vi "neuKLEIN.vi"() -> ()   [LabVIEW 2016] (continued)
  in  "Red 88 Waveform Graph":waveform(dbl)[](graph)=[{"t0"=timestamp(0 s since 1904-01-01), "dt"=0.0001220703125, "Y"=array[4095 elements]}, {"t0"=timestamp(0 s since 1904-01-01), "dt"=0.0001220703125, "Y"=array[4095 elements]}, {"t0"=timestamp(0 s since 1904-01-01), "dt"=0.0001220703125, "Y"=array[4095 elements]}, {"t0"=timestamp(0 s since 1904-01-01), "dt"=0.0001220703125, "Y"=array[4095 elements]}]
  in  "Red MOT 88 Inputs":T21={"Active Device"="6733_Red_88", "Active Channels"=[TRUE, TRUE, TRUE, TRUE, FALSE, FALSE, FALSE, FALSE], "Waveform Parameters"=[[{"Function"=enum."Polynomial", "Initial"=-1.25, "Final"=-0.6, "Degree"=1.0, "Nickname"="Center Freq. [MHz] (0)", "Conversion"=enum."Red Boson Cntr Freq (MHz)", "Constant"=-81.284}, {"Function"=enum."Polynomial", "Initial"=-0.6, "Final"=-0.225, "Degree"=1.0, "Nickname"="(0)", "Conversion"=enum."Red Boson Cntr Freq (MHz)", "Constant"=-81.284}, {"Function"=enum."Polynomial", "Initial"=5.0, "Final"=5.0, "Degree"=1.0, "Nickname"="(0)", "Conversion"=enum."Red Boson Cntr Freq (MHz)", "Constant"=-81.284}, {"Function"=enum."Exponential", "Initial"=1.0, "Final"=0.0, "Degree"=1.0, "Nickname"="", "Conversion"=enum."B Field Grad (G/cm)", "Constant"=0.0}], [{"Function"=enum."Polynomial", "Initial"=1000.0, "Final"=550.0, "Degree"=1.0, "Nickname"="Dither Amp. [kHz] (1)", "Conversion"=enum."Red Boson Dither Amp (kHz)", "Constant"=0.0}, {"Function"=enum."Polynomial", "Initial"=550.0, "Final"=100.0, "Degree"=1.0, "Nickname"="(1)", "Conversion"=enum."Red Boson Dither Amp (kHz)", "Constant"=0.0}, {"Function"=enum."Polynomial", "Initial"=0.0, "Final"=0.0, "Degree"=1.0, "Nickname"="(1)", "Conversion"=enum."Red Boson Dither Amp (kHz)", "Constant"=0.0}, {"Function"=enum."Exponential", "Initial"=0.0, "Final"=0.0, "Degree"=1.0, "Nickname"="", "Conversion"=enum."B Field Grad (G/cm)", "Constant"=0.0}], [{"Function"=enum."Polynomial", "Initial"=10.0, "Final"=10.0, "Degree"=1.0, "Nickname"="Red Boson Power {mW} (2)", "Conversion"=enum."Red Boson Power (mW)", "Constant"=0.0}, {"Function"=enum."Polynomial", "Initial"=10.0, "Final"=5.0, "Degree"=1.0, "Nickname"="(2)", "Conversion"=enum."Red Boson Power (mW)", "Constant"=0.0}, {"Function"=enum."Exponential", "Initial"=5.0, "Final"=0.25, "Degree"=1.0, "Nickname"="(2)", "Conversion"=enum."Red Boson Power (mW)", "Constant"=0.0}, {"Function"=enum."Exponential", "Initial"=0.5, "Final"=0.5, "Degree"=1.0, "Nickname"="", "Conversion"=enum."Red Boson Power (mW)", "Constant"=0.0}], [{"Function"=enum."Polynomial", "Initial"=0.1, "Final"=1.0, "Degree"=1.0, "Nickname"="Red B-Field Grad [G/cm] (3)", "Conversion"=enum."B Field Grad (G/cm)", "Constant"=0.0}, {"Function"=enum."Polynomial", "Initial"=1.0, "Final"=2.0, "Degree"=1.0, "Nickname"="(3)", "Conversion"=enum."B Field Grad (G/cm)", "Constant"=0.0}, {"Function"=enum."Polynomial", "Initial"=2.0, "Final"=2.0, "Degree"=1.0, "Nickname"="(3)", "Conversion"=enum."B Field Grad (G/cm)", "Constant"=0.0}, {"Function"=enum."Exponential", "Initial"=0.2, "Final"=0.2, "Degree"=1.0, "Nickname"="", "Conversion"=enum."B Field Grad (G/cm)", "Constant"=0.0}], [{"Function"=enum."Constant", "Initial"=0.0, "Final"=0.0, "Degree"=1.0, "Nickname"="UNRELIABLE", "Conversion"=enum."Volts", "Constant"=0.0}, {"Function"=enum."Constant", "Initial"=0.0, "Final"=0.0, "Degree"=1.0, "Nickname"="(4)", "Conversion"=enum."Volts", "Constant"=0.0}, {"Function"=enum."Constant", "Initial"=0.0, "Final"=0.0, "Degree"=1.0, "Nickname"="(4)", "Conversion"=enum."Volts", "Constant"=0.0}, {"Function"=enum."Exponential", "Initial"=0.0, "Final"=0.0, "Degree"=1.0, "Nickname"="", "Conversion"=enum."B Field Grad (G/cm)", "Constant"=0.0}], [{"Function"=enum."Constant", "Initial"=0.0, "Final"=0.0, "Degree"=1.0, "Nickname"="Unassigned", "Conversion"=enum."Volts", "Constant"=0.0}, {"Function"=enum."Constant", "Initial"=0.0, "Final"=0.0, "Degree"=1.0, "Nickname"="(5)", "Conversion"=enum."Volts", "Constant"=0.0}, {"Function"=enum."Constant", "Initial"=0.0, "Final"=0.0, "Degree"=1.0, "Nickname"="(5)", "Conversion"=enum."Volts", "Constant"=0.0}, {"Function"=enum."Exponential", "Initial"=0.0, "Final"=0.0, "Degree"=1.0, "Nickname"="", "Conversion"=enum."B Field Grad (G/cm)", "Constant"=0.0}], [{"Function"=enum."Constant", "Initial"=0.0, "Final"=0.0, "Degree"=1.0, "Nickname"="Unassigned", "Conversion"=enum."Volts", "Constant"=0.0}, {"Function"=enum."Constant", "Initial"=0.0, "Final"=0.0, "Degree"=1.0, "Nickname"="(6)", "Conversion"=enum."Volts", "Constant"=0.0}, {"Function"=enum."Constant", "Initial"=0.0, "Final"=0.0, "Degree"=1.0, "Nickname"="(6)", "Conversion"=enum."Volts", "Constant"=0.0}, {"Function"=enum."Exponential", "Initial"=0.0, "Final"=0.0, "Degree"=1.0, "Nickname"="", "Conversion"=enum."B Field Grad (G/cm)", "Constant"=0.0}], [{"Function"=enum."Constant", "Initial"=0.0, "Final"=0.0, "Degree"=1.0, "Nickname"="Unassigned", "Conversion"=enum."Volts", "Constant"=0.0}, {"Function"=enum."Constant", "Initial"=0.0, "Final"=0.0, "Degree"=1.0, "Nickname"="(7)", "Conversion"=enum."Volts", "Constant"=0.0}, {"Function"=enum."Constant", "Initial"=0.0, "Final"=0.0, "Degree"=1.0, "Nickname"="(7)", "Conversion"=enum."Volts", "Constant"=0.0}, {"Function"=enum."Exponential", "Initial"=0.0, "Final"=0.0, "Degree"=1.0, "Nickname"="", "Conversion"=enum."B Field Grad (G/cm)", "Constant"=0.0}]], "Active Phases"=[TRUE, TRUE, TRUE, FALSE, FALSE, FALSE], "Phase Times"=[0.15, 0.25, 0.1, 0.05], "Trigger Channel"="/6733_Red_88/PFI3"} {"Phase Times" format="%.0p"; "Waveform Parameters"."Degree" min=1.0}
  in  "Red MOT 87 Notes":string="NOTES:\nChannel 0 - Red 87 Trap Center Freq.\nAs of 2017.05.17 Slave 2 (87 trapping slave) is injection locked -82 MHz of the 3P1 F=11/2 transition. \n\nChannel 4 - Red 87 Stir Center Freq\nAs of 2017.05.17, Slave 1 (87 Stir Slave) is injection locked -143.71 MHz of the 3P1 F=9/2 transition\n\n\n2018.07.12\nThere is an absolute offset to the calibration used in the Labview program to calculate the voltage for a certain freq out of the VCOs and the actual freq the VCO  outputs.  I compensate for this descrepancy by measurnig what input corresponds to the output I want. While absolute freq value has an offset, the slope of the calibration is pretty good so detuning by a certain amount is fairly accurate. Actual was measured out of the Aux port on the VCO's and set is what you program into the constant value for each channel.\nTrap:- Actual: +82 MHz, Set: +81.67 MHz\nStir:- Actual: +143.71 MHz, Set: +144.187 MHz\n"
  in  "Red 87 Waveform Graph":waveform(dbl)[](graph)=[{"t0"=timestamp(0 s since 1904-01-01), "dt"=0.00016479894528675015, "Y"=array[2730 elements]}, {"t0"=timestamp(0 s since 1904-01-01), "dt"=0.00016479894528675015, "Y"=array[2730 elements]}, {"t0"=timestamp(0 s since 1904-01-01), "dt"=0.00016479894528675015, "Y"=array[2730 elements]}, {"t0"=timestamp(0 s since 1904-01-01), "dt"=0.00016479894528675015, "Y"=array[2730 elements]}, {"t0"=timestamp(0 s since 1904-01-01), "dt"=0.00016479894528675015, "Y"=array[2730 elements]}, {"t0"=timestamp(0 s since 1904-01-01), "dt"=0.00016479894528675015, "Y"=array[2730 elements]}]
  in  "Red MOT 87 Inputs":T21={"Active Device"="6733_Red_87", "Active Channels"=[TRUE, TRUE, TRUE, FALSE, TRUE, TRUE, TRUE, FALSE], "Waveform Parameters"=[[{"Function"=enum."Polynomial", "Initial"=-1.2, "Final"=-0.75, "Degree"=1.0, "Nickname"="87 Trap Center Freq [MHz]", "Conversion"=enum."Red 87 Trap Cntr Freq (MHz)", "Constant"=81.67}, {"Function"=enum."Polynomial", "Initial"=-0.75, "Final"=-0.3, "Degree"=1.0, "Nickname"="(0)", "Conversion"=enum."Red 87 Trap Cntr Freq (MHz)", "Constant"=81.67}, {"Function"=enum."Polynomial", "Initial"=5.0, "Final"=5.0, "Degree"=1.0, "Nickname"="(0)", "Conversion"=enum."Red 87 Trap Cntr Freq (MHz)", "Constant"=81.67}, {"Function"=enum."Polynomial", "Initial"=-0.4, "Final"=-0.4, "Degree"=1.0, "Nickname"="(0)", "Conversion"=enum."Red 87 Trap Cntr Freq (MHz)", "Constant"=81.67}], [{"Function"=enum."Polynomial", "Initial"=1000.0, "Final"=600.0, "Degree"=1.0, "Nickname"="87 Trap Dither Amp [kHz]", "Conversion"=enum."Red 87 Trap Dither Amp (kHz)", "Constant"=0.0}, {"Function"=enum."Polynomial", "Initial"=600.0, "Final"=275.0, "Degree"=1.0, "Nickname"="(1)", "Conversion"=enum."Red 87 Trap Dither Amp (kHz)", "Constant"=0.0}, {"Function"=enum."Polynomial", "Initial"=0.0, "Final"=0.0, "Degree"=1.0, "Nickname"="(1)", "Conversion"=enum."Red 87 Trap Dither Amp (kHz)", "Constant"=0.0}, {"Function"=enum."Polynomial", "Initial"=200.0, "Final"=200.0, "Degree"=1.0, "Nickname"="(1)", "Conversion"=enum."Red 87 Trap Dither Amp (kHz)", "Constant"=0.0}], [{"Function"=enum."Polynomial", "Initial"=14.0, "Final"=14.0, "Degree"=1.0, "Nickname"="87 Trap Power [mW]", "Conversion"=enum."Red 87 Trap Power (mW)", "Constant"=0.0}, {"Function"=enum."Polynomial", "Initial"=14.0, "Final"=5.0, "Degree"=1.0, "Nickname"="(2)", "Conversion"=enum."Red 87 Trap Power (mW)", "Constant"=0.0}, {"Function"=enum."Exponential", "Initial"=3.0, "Final"=0.05, "Degree"=1.0, "Nickname"="(2)", "Conversion"=enum."Red 87 Trap Power (mW)", "Constant"=0.0}, {"Function"=enum."Polynomial", "Initial"=14.0, "Final"=14.0, "Degree"=1.0, "Nickname"="(2)", "Conversion"=enum."Red 87 Trap Power (mW)", "Constant"=0.0}], [{"Function"=enum."Constant", "Initial"=0.0, "Final"=0.0, "Degree"=1.0, "Nickname"="Unassigned", "Conversion"=enum."Volts", "Constant"=0.0}, {"Function"=enum."Constant", "Initial"=0.0, "Final"=0.0, "Degree"=1.0, "Nickname"="(3)", "Conversion"=enum."Volts", "Constant"=0.0}, {"Function"=enum."Constant", "Initial"=0.0, "Final"=0.0, "Degree"=1.0, "Nickname"="(3)", "Conversion"=enum."Volts", "Constant"=0.0}, {"Function"=enum."Constant", "Initial"=0.0, "Final"=0.0, "Degree"=1.0, "Nickname"="(3)", "Conversion"=enum."Volts", "Constant"=0.0}], [{"Function"=enum."Polynomial", "Initial"=-1.1, "Final"=-0.9, "Degree"=1.0, "Nickname"="87 Stir Center Freq {MHz}", "Conversion"=enum."Red 87 Stir Cntr Freq (MHz)", "Constant"=144.187}, {"Function"=enum."Polynomial", "Initial"=-0.9, "Final"=-0.4, "Degree"=1.0, "Nickname"="(4)", "Conversion"=enum."Red 87 Stir Cntr Freq (MHz)", "Constant"=144.187}, {"Function"=enum."Polynomial", "Initial"=5.0, "Final"=5.0, "Degree"=1.0, "Nickname"="(4)", "Conversion"=enum."Red 87 Stir Cntr Freq (MHz)", "Constant"=144.187}, {"Function"=enum."Polynomial", "Initial"=-0.5, "Final"=-0.5, "Degree"=1.0, "Nickname"="(4)", "Conversion"=enum."Red 87 Stir Cntr Freq (MHz)", "Constant"=144.187}], [{"Function"=enum."Polynomial", "Initial"=1000.0, "Final"=650.0, "Degree"=1.0, "Nickname"="87 Stir Dither Amp [kHz]", "Conversion"=enum."Red 87 Stir Dither Amp (kHz)", "Constant"=0.0}, {"Function"=enum."Polynomial", "Initial"=650.0, "Final"=150.0, "Degree"=1.0, "Nickname"="(5)", "Conversion"=enum."Red 87 Stir Dither Amp (kHz)", "Constant"=0.0}, {"Function"=enum."Polynomial", "Initial"=0.0, "Final"=0.0, "Degree"=1.0, "Nickname"="(5)", "Conversion"=enum."Red 87 Stir Dither Amp (kHz)", "Constant"=0.0}, {"Function"=enum."Polynomial", "Initial"=200.0, "Final"=200.0, "Degree"=1.0, "Nickname"="(5)", "Conversion"=enum."Red 87 Stir Dither Amp (kHz)", "Constant"=0.0}], [{"Function"=enum."Polynomial", "Initial"=19.0, "Final"=19.0, "Degree"=1.0, "Nickname"="87 Stir Power {mW}", "Conversion"=enum."Red 87 Stir Power (mW)", "Constant"=0.0}, {"Function"=enum."Polynomial", "Initial"=19.0, "Final"=19.0, "Degree"=1.0, "Nickname"="(6)", "Conversion"=enum."Red 87 Stir Power (mW)", "Constant"=0.0}, {"Function"=enum."Exponential", "Initial"=0.5, "Final"=0.05, "Degree"=1.0, "Nickname"="(6)", "Conversion"=enum."Red 87 Stir Power (mW)", "Constant"=0.0}, {"Function"=enum."Polynomial", "Initial"=19.0, "Final"=19.0, "Degree"=1.0, "Nickname"="(6)", "Conversion"=enum."Red 87 Stir Power (mW)", "Constant"=0.0}], [{"Function"=enum."Constant", "Initial"=0.0, "Final"=0.0, "Degree"=1.0, "Nickname"="Unassigned", "Conversion"=enum."Volts", "Constant"=0.0}, {"Function"=enum."Constant", "Initial"=0.0, "Final"=0.0, "Degree"=1.0, "Nickname"="(7)", "Conversion"=enum."Volts", "Constant"=0.0}, {"Function"=enum."Constant", "Initial"=0.0, "Final"=0.0, "Degree"=1.0, "Nickname"="(7)", "Conversion"=enum."Volts", "Constant"=0.0}, {"Function"=enum."Constant", "Initial"=0.0, "Final"=0.0, "Degree"=1.0, "Nickname"="(7)", "Conversion"=enum."Volts", "Constant"=0.0}]], "Active Phases"=[TRUE, TRUE, TRUE, FALSE, FALSE, FALSE], "Phase Times"=[0.15, 0.25, 0.05, 0.05], "Trigger Channel"="/6733_Red_87/PFI6"} {"Phase Times" format="%.0p"; "Waveform Parameters"."Degree" min=1.0}
  in  "ODT Waveform Graph":waveform(dbl)[](graph)=[{"t0"=timestamp(0 s since 1904-01-01), "dt"=1.2208521548040533e-05, "Y"=array[4095 elements]}, {"t0"=timestamp(0 s since 1904-01-01), "dt"=1.2208521548040533e-05, "Y"=array[4095 elements]}]
  in  "ODT Params":T25={"Waveform Parameters"=[[{"Initial Value"=-9.25, "Final Value"=-10.0, "Tau"=0.0, "Eta"=1.0, "Nickname"="Loading Trap  A", "Function Type"=enum."Power Law", "Conversion"=enum."Volts", "Constant"=-9.25}, {"Initial Value"=-9.25, "Final Value"=-9.25, "Tau"=inf, "Eta"=10.0, "Nickname"="Loading Trap  B", "Function Type"=enum."Evap - Calc Tau", "Conversion"=enum."Volts", "Constant"=0.0}, {"Initial Value"=-9.25, "Final Value"=-9.25, "Tau"=0.0, "Eta"=1.0, "Nickname"="Loading Trap  C", "Function Type"=enum."Power Law", "Conversion"=enum."Volts", "Constant"=-9.25}, {"Initial Value"=-9.25, "Final Value"=-4.2, "Tau"=9.638407328580247, "Eta"=10.0, "Nickname"="Loading Trap  D", "Function Type"=enum."Evap - Calc Tau", "Conversion"=enum."Volts", "Constant"=0.0}], [{"Initial Value"=-0.75, "Final Value"=-1.4479531262021905, "Tau"=0.0, "Eta"=1.0, "Nickname"="Sheet/Dimple Trap A", "Function Type"=enum."Power Law", "Conversion"=enum."Volts", "Constant"=-0.75}, {"Initial Value"=-0.75, "Final Value"=-0.75, "Tau"=0.0, "Eta"=0.5, "Nickname"="Sheet/Dimple Trap B", "Function Type"=enum."Power Law", "Conversion"=enum."Volts", "Constant"=-0.75}, {"Initial Value"=-0.75, "Final Value"=-0.75, "Tau"=0.0, "Eta"=1.0, "Nickname"="Sheet/Dimple Trap C", "Function Type"=enum."Power Law", "Conversion"=enum."Volts", "Constant"=-0.75}, {"Initial Value"=-0.75, "Final Value"=-0.75, "Tau"=0.0, "Eta"=1.0, "Nickname"="Sheet/Dimple Trap D", "Function Type"=enum."Power Law", "Conversion"=enum."Volts", "Constant"=-0.75}]], "Active Phases"=[TRUE, FALSE, FALSE, FALSE], "Active Channels"=[TRUE, TRUE], "Phase Times (s)"=[0.05, 3.0, 0.55, 7.0], "Active Device"="6221_IR_ODT", "Trigger Channel"="/6221_IR_ODT/PFI0", "Evaporation Phase"=1.0, "Evaporation Channel"=0.0} {"Evaporation Channel" min=0.0 max=1.0 step=1.0; "Evaporation Phase" min=0.0 max=4.0 step=1.0; "Phase Times (s)" format="%#_6p"}
  in  "Green Lattice Waveform Graph":waveform(dbl)[](graph)=[{"t0"=timestamp(0 s since 1904-01-01), "dt"=1.2208521548040533e-05, "Y"=array[4095 elements]}, {"t0"=timestamp(0 s since 1904-01-01), "dt"=1.2208521548040533e-05, "Y"=array[4095 elements]}]
  in  "6229 Green Lattice Inputs":T28={"Active Device"="6229_Green_Lattice", "Active Channels"=[TRUE, TRUE, FALSE, FALSE], "Active Phases"=[TRUE, FALSE, FALSE, FALSE, FALSE, FALSE], "Phase Times"=[0.05, 4.0, 0.5, 3.1], "Trigger Channel"="/6229_Green_Lattice/PFI0", "FIFO Buffer Size"=8191.0, "Sample Step Time (us)"=12.208521548040533, "Initialization Parameters"={"Enable Initialization"=TRUE, "Initial Values"=[0.1, 0.1, 0.1, 0.0]}, "Waveform Parameters"=[[{"Initial Value"=0.0, "Final Value"=0.0, "Tau"=0.0, "Eta"=1.0, "Nickname"="Arm A - Phase 0", "Function Type"=enum."Constant", "Conversion"=enum."Volts", "Constant"=8.25}, {"Initial Value"=8.25, "Final Value"=0.0, "Tau"=0.0, "Eta"=6.0, "Nickname"="Arm A - Phase 1", "Function Type"=enum."Constant", "Conversion"=enum."Volts", "Constant"=0.0}, {"Initial Value"=2.5, "Final Value"=0.0, "Tau"=0.0, "Eta"=0.0, "Nickname"="Arm A - Phase 2", "Function Type"=enum."Constant", "Conversion"=enum."Volts", "Constant"=0.0}, {"Initial Value"=2.0, "Final Value"=3.5416846293181257, "Tau"=0.0, "Eta"=1.0, "Nickname"="", "Function Type"=enum."Power Law", "Conversion"=enum."Volts", "Constant"=8.5}, {"Initial Value"=0.0, "Final Value"=0.0, "Tau"=0.0, "Eta"=0.0, "Nickname"="", "Function Type"=enum."Constant", "Conversion"=enum."Volts", "Constant"=0.0}, {"Initial Value"=0.0, "Final Value"=0.0, "Tau"=0.0, "Eta"=0.0, "Nickname"="", "Function Type"=enum."Constant", "Conversion"=enum."Volts", "Constant"=0.0}], [{"Initial Value"=0.0, "Final Value"=0.0, "Tau"=0.0, "Eta"=1.0, "Nickname"="Arm B - Phase 0", "Function Type"=enum."Constant", "Conversion"=enum."Volts", "Constant"=7.75}, {"Initial Value"=8.0, "Final Value"=7.0, "Tau"=30.301092759110453, "Eta"=6.0, "Nickname"="Arm B - Phase 1", "Function Type"=enum."Evap - Calc Tau", "Conversion"=enum."Volts", "Constant"=0.0}, {"Initial Value"=4.5, "Final Value"=3.0, "Tau"=0.0, "Eta"=0.0, "Nickname"="Arm B - Phase 2", "Function Type"=enum."Constant", "Conversion"=enum."Volts", "Constant"=0.0}, {"Initial Value"=2.0, "Final Value"=1.6181503373960489, "Tau"=0.0, "Eta"=1.0, "Nickname"="", "Function Type"=enum."Power Law", "Conversion"=enum."Volts", "Constant"=2.8}, {"Initial Value"=0.0, "Final Value"=0.0, "Tau"=0.0, "Eta"=0.0, "Nickname"="", "Function Type"=enum."Constant", "Conversion"=enum."Volts", "Constant"=0.0}, {"Initial Value"=0.0, "Final Value"=0.0, "Tau"=0.0, "Eta"=0.0, "Nickname"="", "Function Type"=enum."Constant", "Conversion"=enum."Volts", "Constant"=0.0}], [{"Initial Value"=0.0, "Final Value"=0.0, "Tau"=0.0, "Eta"=0.0, "Nickname"="Arm C - Phase 0", "Function Type"=enum."Constant", "Conversion"=enum."Volts", "Constant"=0.0}, {"Initial Value"=0.0, "Final Value"=0.0, "Tau"=0.0, "Eta"=1.0, "Nickname"="Arm C - Phase 1", "Function Type"=enum."Constant", "Conversion"=enum."Volts", "Constant"=0.0}, {"Initial Value"=0.0, "Final Value"=6.0, "Tau"=0.0, "Eta"=1.0, "Nickname"="Arm C - Phase 2", "Function Type"=enum."Power Law", "Conversion"=enum."Volts", "Constant"=0.0}, {"Initial Value"=2.0, "Final Value"=0.0, "Tau"=0.0, "Eta"=1.0, "Nickname"="", "Function Type"=enum."Power Law", "Conversion"=enum."Volts", "Constant"=0.0}, {"Initial Value"=0.0, "Final Value"=0.0, "Tau"=0.0, "Eta"=0.0, "Nickname"="", "Function Type"=enum."Constant", "Conversion"=enum."Volts", "Constant"=0.0}, {"Initial Value"=0.0, "Final Value"=0.0, "Tau"=0.0, "Eta"=0.0, "Nickname"="", "Function Type"=enum."Constant", "Conversion"=enum."Volts", "Constant"=0.0}], [{"Initial Value"=2.0, "Final Value"=1.75, "Tau"=0.9, "Eta"=1.0, "Nickname"="", "Function Type"=enum."Power Law", "Conversion"=enum."Volts", "Constant"=0.0}, {"Initial Value"=2.0, "Final Value"=0.0, "Tau"=0.0, "Eta"=1.0, "Nickname"="", "Function Type"=enum."Power Law", "Conversion"=enum."Volts", "Constant"=0.0}, {"Initial Value"=0.0, "Final Value"=3.0, "Tau"=0.2, "Eta"=1.0, "Nickname"="", "Function Type"=enum."Power Law", "Conversion"=enum."Volts", "Constant"=0.0}, {"Initial Value"=2.0, "Final Value"=0.0, "Tau"=0.0, "Eta"=1.0, "Nickname"="", "Function Type"=enum."Power Law", "Conversion"=enum."Volts", "Constant"=0.2}, {"Initial Value"=1.0, "Final Value"=0.0, "Tau"=0.0, "Eta"=1.0, "Nickname"="", "Function Type"=enum."Power Law", "Conversion"=enum."B Field Grad (G/cm)", "Constant"=0.0}, {"Initial Value"=1.0, "Final Value"=0.0, "Tau"=0.0, "Eta"=1.0, "Nickname"="", "Function Type"=enum."Power Law", "Conversion"=enum."B Field Grad (G/cm)", "Constant"=0.0}]]} {"Phase Times" format="%_3p"}
  in  "FPGA_panel_tab_ctrl":enum32{"Control", "Labels"}(tab)
  in  "FPGA_cntrl":T30={"Channel 0"={"Operation"=0, "Input A"=32, "Output - LO"=0.0, "Output - HI"=0.0, "Inputs"=[32, 32, 32, 32], "Output Values"=[0.0, 0.0, 0.0, 0.0, 0.0], "Num. Inputs"=0, "Set Point"=0.0, "Inv."=[FALSE, FALSE, FALSE, FALSE], "Inv. A"=FALSE, "Inv. B"=FALSE, "Input B"=32}, "Channel 1"={"Operation"=0, "Input A"=32, "Output - LO"=0.0, "Output - HI"=0.0, "Inputs"=[0, 0, 0, 0], "Output Values"=[0.0, 0.0, 0.0, 0.0, 0.0], "Num. Inputs"=0, "Set Point"=0.0, "Inv."=[FALSE, FALSE, FALSE, FALSE], "Inv. A"=FALSE, "Inv. B"=FALSE, "Input B"=32}, "Channel 2"={"Operation"=1, "Input A"=32, "Output - LO"=0.0, "Output - HI"=0.0, "Inputs"=[0, 0, 0, 0], "Output Values"=[0.0, 0.0, 0.0, 0.0, 0.0], "Num. Inputs"=4, "Set Point"=4.20001220703125, "Inv."=[FALSE, FALSE, FALSE, FALSE], "Inv. A"=FALSE, "Inv. B"=FALSE, "Input B"=32}, "Channel 3"={"Operation"=4, "Input A"=5, "Output - LO"=0.0, "Output - HI"=4.0, "Inputs"=[0, 0, 0, 0], "Output Values"=[0.0, 0.0, 0.0, 0.0, 0.0], "Num. Inputs"=4, "Set Point"=0.0, "Inv."=[FALSE, FALSE, FALSE, FALSE], "Inv. A"=FALSE, "Inv. B"=FALSE, "Input B"=6}, "Channel 4"={"Operation"=2, "Input A"=7, "Output - LO"=-0.149993896484375, "Output - HI"=-0.20001220703125, "Inputs"=[0, 0, 0, 0], "Output Values"=[0.0, 0.0, 0.0, 0.0, 0.0], "Num. Inputs"=4, "Set Point"=-0.1099853515625, "Inv."=[FALSE, FALSE, FALSE, FALSE], "Inv. A"=FALSE, "Inv. B"=FALSE, "Input B"=32}, "Channel 5"={"Operation"=2, "Input A"=7, "Output - LO"=1.579986572265625, "Output - HI"=1.29998779296875, "Inputs"=[0, 0, 0, 0], "Output Values"=[0.0, 0.0, 0.0, 0.0, 0.0], "Num. Inputs"=4, "Set Point"=1.5, "Inv."=[FALSE, FALSE, FALSE, FALSE], "Inv. A"=FALSE, "Inv. B"=FALSE, "Input B"=32}, "Channel 6"={"Operation"=2, "Input A"=7, "Output - LO"=1.260009765625, "Output - HI"=2.0, "Inputs"=[7, 9, 0, 0], "Output Values"=[1.209991455078125, 10.0, 1.165008544921875, 0.0, 0.0], "Num. Inputs"=2, "Set Point"=1.125, "Inv."=[TRUE, TRUE, FALSE, FALSE], "Inv. A"=FALSE, "Inv. B"=FALSE, "Input B"=32}, "Channel 7"={"Operation"=2, "Input A"=8, "Output - LO"=0.95001220703125, "Output - HI"=1.75, "Inputs"=[0, 0, 0, 0], "Output Values"=[0.0, 0.0, 0.0, 0.0, 0.0], "Num. Inputs"=4, "Set Point"=1.75, "Inv."=[FALSE, FALSE, FALSE, FALSE], "Inv. A"=FALSE, "Inv. B"=FALSE, "Input B"=32}, "Channel 8"={"Operation"=6, "Input A"=32, "Output - LO"=0.0, "Output - HI"=0.0, "Inputs"=[0, 1, 32, 3], "Output Values"=[-5.29998779296875, -1.850006103515625, 0.0, -5.399993896484375, -1.959991455078125], "Num. Inputs"=4, "Set Point"=7.75, "Inv."=[FALSE, FALSE, TRUE, TRUE], "Inv. A"=FALSE, "Inv. B"=FALSE, "Input B"=32}, "Channel 9"={"Operation"=2, "Input A"=2, "Output - LO"=-0.29998779296875, "Output - HI"=-5.5, "Inputs"=[0, 0, 0, 0], "Output Values"=[0.0, 0.0, 0.0, 0.0, 0.0], "Num. Inputs"=0, "Set Point"=0.0, "Inv."=[FALSE, FALSE, FALSE, FALSE], "Inv. A"=FALSE, "Inv. B"=FALSE, "Input B"=32}, "Channel 10"={"Operation"=0, "Input A"=32, "Output - LO"=0.0, "Output - HI"=0.0, "Inputs"=[0, 0, 0, 0], "Output Values"=[0.0, 0.0, 0.0, 0.0, 0.0], "Num. Inputs"=4, "Set Point"=0.0, "Inv."=[FALSE, FALSE, FALSE, FALSE], "Inv. A"=FALSE, "Inv. B"=FALSE, "Input B"=32}, "Channel 11"={"Operation"=0, "Input A"=32, "Output - LO"=0.0, "Output - HI"=0.0, "Inputs"=[0, 0, 0, 0], "Output Values"=[0.0, 0.0, 0.0, 0.0, 0.0], "Num. Inputs"=4, "Set Point"=0.0, "Inv."=[FALSE, FALSE, FALSE, FALSE], "Inv. A"=FALSE, "Inv. B"=FALSE, "Input B"=32}, "Channel 12"={"Operation"=0, "Input A"=32, "Output - LO"=0.0, "Output - HI"=0.0, "Inputs"=[0, 0, 0, 0], "Output Values"=[0.0, 0.0, 0.0, 0.0, 0.0], "Num. Inputs"=4, "Set Point"=0.0, "Inv."=[FALSE, FALSE, FALSE, FALSE], "Inv. A"=FALSE, "Inv. B"=FALSE, "Input B"=32}, "Channel 13"={"Operation"=0, "Input A"=32, "Output - LO"=0.0, "Output - HI"=0.0, "Inputs"=[0, 0, 0, 0], "Output Values"=[0.0, 0.0, 0.0, 0.0, 0.0], "Num. Inputs"=4, "Set Point"=0.0, "Inv."=[FALSE, FALSE, FALSE, FALSE], "Inv. A"=FALSE, "Inv. B"=FALSE, "Input B"=32}, "Channel 14"={"Operation"=0, "Input A"=32, "Output - LO"=0.0, "Output - HI"=0.0, "Inputs"=[0, 0, 0, 0], "Output Values"=[0.0, 0.0, 0.0, 0.0, 0.0], "Num. Inputs"=4, "Set Point"=0.0, "Inv."=[FALSE, FALSE, FALSE, FALSE], "Inv. A"=FALSE, "Inv. B"=FALSE, "Input B"=32}, "Channel 15"={"Operation"=0, "Input A"=32, "Output - LO"=0.0, "Output - HI"=0.0, "Inputs"=[0, 0, 0, 0], "Output Values"=[0.0, 0.0, 0.0, 0.0, 0.0], "Num. Inputs"=4, "Set Point"=0.0, "Inv."=[FALSE, FALSE, FALSE, FALSE], "Inv. A"=FALSE, "Inv. B"=FALSE, "Input B"=32}} {"Channel 15"."Input B" items=["DIO0", "DIO1", "DIO2", "DIO3", "DIO4", "DIO5", "DIO6", "DIO7", "DIO8", "DIO9", "DIO10", "DIO11", "DIO12", "DIO13", "DIO14", "DIO15", "DIO16", "DIO17", "DIO18", "DIO19", "DIO20", "DIO21", "DIO22", "DIO23", "DIO24", "DIO25", "DIO26", "DIO27", "DIO28", "DIO29", "DIO30", "DIO31", "FALSE"]; "Channel 15"."Input A" items=["DIO0", "DIO1", "DIO2", "DIO3", "DIO4", "DIO5", "DIO6", "DIO7", "DIO8", "DIO9", "DIO10", "DIO11", "DIO12", "DIO13", "DIO14", "DIO15", "DIO16", "DIO17", "DIO18", "DIO19", "DIO20", "DIO21", "DIO22", "DIO23", "DIO24", "DIO25", "DIO26", "DIO27", "DIO28", "DIO29", "DIO30", "DIO31", "FALSE"]; "Channel 15"."Inputs" items=["DIO0", "DIO1", "DIO2", "DIO3", "DIO4", "DIO5", "DIO6", "DIO7", "DIO8", "DIO9", "DIO10", "DIO11", "DIO12", "DIO13", "DIO14", "DIO15", "DIO16", "DIO17", "DIO18", "DIO19", "DIO20", "DIO21", "DIO22", "DIO23", "DIO24", "DIO25", "DIO26", "DIO27", "DIO28", "DIO29", "DIO30", "DIO31", "FALSE"]; "Channel 15"."Operation" items=["OFF", "Constant", "Bool - Basic Switch", "Bool - AND Switch", "Bool - OR Switch", "Custom - Comp Basic Switch", "Custom - 461nm Freq."]; "Channel 14"."Input B" items=["DIO0", "DIO1", "DIO2", "DIO3", "DIO4", "DIO5", "DIO6", "DIO7", "DIO8", "DIO9", "DIO10", "DIO11", "DIO12", "DIO13", "DIO14", "DIO15", "DIO16", "DIO17", "DIO18", "DIO19", "DIO20", "DIO21", "DIO22", "DIO23", "DIO24", "DIO25", "DIO26", "DIO27", "DIO28", "DIO29", "DIO30", "DIO31", "FALSE"]; "Channel 14"."Input A" items=["DIO0", "DIO1", "DIO2", "DIO3", "DIO4", "DIO5", "DIO6", "DIO7", "DIO8", "DIO9", "DIO10", "DIO11", "DIO12", "DIO13", "DIO14", "DIO15", "DIO16", "DIO17", "DIO18", "DIO19", "DIO20", "DIO21", "DIO22", "DIO23", "DIO24", "DIO25", "DIO26", "DIO27", "DIO28", "DIO29", "DIO30", "DIO31", "FALSE"]; "Channel 14"."Inputs" items=["DIO0", "DIO1", "DIO2", "DIO3", "DIO4", "DIO5", "DIO6", "DIO7", "DIO8", "DIO9", "DIO10", "DIO11", "DIO12", "DIO13", "DIO14", "DIO15", "DIO16", "DIO17", "DIO18", "DIO19", "DIO20", "DIO21", "DIO22", "DIO23", "DIO24", "DIO25", "DIO26", "DIO27", "DIO28", "DIO29", "DIO30", "DIO31", "FALSE"]; "Channel 14"."Operation" items=["OFF", "Constant", "Bool - Basic Switch", "Bool - AND Switch", "Bool - OR Switch", "Custom - Comp Basic Switch", "Custom - 461nm Freq."]; "Channel 13"."Input B" items=["DIO0", "DIO1", "DIO2", "DIO3", "DIO4", "DIO5", "DIO6", "DIO7", "DIO8", "DIO9", "DIO10", "DIO11", "DIO12", "DIO13", "DIO14", "DIO15", "DIO16", "DIO17", "DIO18", "DIO19", "DIO20", "DIO21", "DIO22", "DIO23", "DIO24", "DIO25", "DIO26", "DIO27", "DIO28", "DIO29", "DIO30", "DIO31", "FALSE"]; "Channel 13"."Input A" items=["DIO0", "DIO1", "DIO2", "DIO3", "DIO4", "DIO5", "DIO6", "DIO7", "DIO8", "DIO9", "DIO10", "DIO11", "DIO12", "DIO13", "DIO14", "DIO15", "DIO16", "DIO17", "DIO18", "DIO19", "DIO20", "DIO21", "DIO22", "DIO23", "DIO24", "DIO25", "DIO26", "DIO27", "DIO28", "DIO29", "DIO30", "DIO31", "FALSE"]; "Channel 13"."Inputs" items=["DIO0", "DIO1", "DIO2", "DIO3", "DIO4", "DIO5", "DIO6", "DIO7", "DIO8", "DIO9", "DIO10", "DIO11", "DIO12", "DIO13", "DIO14", "DIO15", "DIO16", "DIO17", "DIO18", "DIO19", "DIO20", "DIO21", "DIO22", "DIO23", "DIO24", "DIO25", "DIO26", "DIO27", "DIO28", "DIO29", "DIO30", "DIO31", "FALSE"]; "Channel 13"."Operation" items=["OFF", "Constant", "Bool - Basic Switch", "Bool - AND Switch", "Bool - OR Switch", "Custom - Comp Basic Switch", "Custom - 461nm Freq."]; "Channel 12"."Input B" items=["DIO0", "DIO1", "DIO2", "DIO3", "DIO4", "DIO5", "DIO6", "DIO7", "DIO8", "DIO9", "DIO10", "DIO11", "DIO12", "DIO13", "DIO14", "DIO15", "DIO16", "DIO17", "DIO18", "DIO19", "DIO20", "DIO21", "DIO22", "DIO23", "DIO24", "DIO25", "DIO26", "DIO27", "DIO28", "DIO29", "DIO30", "DIO31", "FALSE"]; "Channel 12"."Input A" items=["DIO0", "DIO1", "DIO2", "DIO3", "DIO4", "DIO5", "DIO6", "DIO7", "DIO8", "DIO9", "DIO10", "DIO11", "DIO12", "DIO13", "DIO14", "DIO15", "DIO16", "DIO17", "DIO18", "DIO19", "DIO20", "DIO21", "DIO22", "DIO23", "DIO24", "DIO25", "DIO26", "DIO27", "DIO28", "DIO29", "DIO30", "DIO31", "FALSE"]; "Channel 12"."Inputs" items=["DIO0", "DIO1", "DIO2", "DIO3", "DIO4", "DIO5", "DIO6", "DIO7", "DIO8", "DIO9", "DIO10", "DIO11", "DIO12", "DIO13", "DIO14", "DIO15", "DIO16", "DIO17", "DIO18", "DIO19", "DIO20", "DIO21", "DIO22", "DIO23", "DIO24", "DIO25", "DIO26", "DIO27", "DIO28", "DIO29", "DIO30", "DIO31", "FALSE"]; "Channel 12"."Operation" items=["OFF", "Constant", "Bool - Basic Switch", "Bool - AND Switch", "Bool - OR Switch", "Custom - Comp Basic Switch", "Custom - 461nm Freq."]; "Channel 11"."Input B" items=["DIO0", "DIO1", "DIO2", "DIO3", "DIO4", "DIO5", "DIO6", "DIO7", "DIO8", "DIO9", "DIO10", "DIO11", "DIO12", "DIO13", "DIO14", "DIO15", "DIO16", "DIO17", "DIO18", "DIO19", "DIO20", "DIO21", "DIO22", "DIO23", "DIO24", "DIO25", "DIO26", "DIO27", "DIO28", "DIO29", "DIO30", "DIO31", "FALSE"]; "Channel 11"."Input A" items=["DIO0", "DIO1", "DIO2", "DIO3", "DIO4", "DIO5", "DIO6", "DIO7", "DIO8", "DIO9", "DIO10", "DIO11", "DIO12", "DIO13", "DIO14", "DIO15", "DIO16", "DIO17", "DIO18", "DIO19", "DIO20", "DIO21", "DIO22", "DIO23", "DIO24", "DIO25", "DIO26", "DIO27", "DIO28", "DIO29", "DIO30", "DIO31", "FALSE"]; "Channel 11"."Inputs" items=["DIO0", "DIO1", "DIO2", "DIO3", "DIO4", "DIO5", "DIO6", "DIO7", "DIO8", "DIO9", "DIO10", "DIO11", "DIO12", "DIO13", "DIO14", "DIO15", "DIO16", "DIO17", "DIO18", "DIO19", "DIO20", "DIO21", "DIO22", "DIO23", "DIO24", "DIO25", "DIO26", "DIO27", "DIO28", "DIO29", "DIO30", "DIO31", "FALSE"]; "Channel 11"."Operation" items=["OFF", "Constant", "Bool - Basic Switch", "Bool - AND Switch", "Bool - OR Switch", "Custom - Comp Basic Switch", "Custom - 461nm Freq."]; "Channel 10"."Input B" items=["DIO0", "DIO1", "DIO2", "DIO3", "DIO4", "DIO5", "DIO6", "DIO7", "DIO8", "DIO9", "DIO10", "DIO11", "DIO12", "DIO13", "DIO14", "DIO15", "DIO16", "DIO17", "DIO18", "DIO19", "DIO20", "DIO21", "DIO22", "DIO23", "DIO24", "DIO25", "DIO26", "DIO27", "DIO28", "DIO29", "DIO30", "DIO31", "FALSE"]; "Channel 10"."Input A" items=["DIO0", "DIO1", 